vi "Dresden R2R Sputter 03.02.2018 IY24.vi"() -> ()   [LabVIEW 2009] (continued)
                                frame #1 {
                                }
                                }
                                }
                                frame #1 {
                                n15923 = local read "Semi"() -> (w27844)
                                n15924 = case shown="False" w27844 {
                                frame #0 {
                                n15925 = local write "Ch1_PA15"(T/1 ("PA3")) -> ()
                                n15926 = Wait Until Next ms Multiple(millisecond multiple=i32? 1000) -> ()  [unwired: 1 out]
                                }
                                frame #1 {
                                }
                                }
                                }
                                }
                              }
                              frame #1 {
                              }
                            }
                          }
                          frame #10 {
                            # "OPEN CH1-VBV"
                            n15927 = local read "Semi"() -> (w27847)
                            n15928 = case shown="False" w27847 {
                              frame #0 {
                                n15929 = stacked-sequence {
                                frame #0 {
                                n15930 = local read "Semi"() -> (w27848)
                                n15931 = case shown="False" w27848 {
                                frame #0 {
                                n15932 = while {
                                i -> [w27855]
                                stop <- w27850 stop-if-true
                                n15933 = Greater?(x=w27855, y=i32? 50) -> (0:w27853)
                                n15934 = case shown="True" w27853 {
                                frame #0 {
                                }
                                frame #1 {
                                n15935 = local write "Semi"(T/1 ("Semi")) -> ()
                                n15936 = local write "Error Message"("Start up process  cancelled\nbecause  CH1-VBV not opened.\nPlease check  CH1-VBV connections." ("Error Message")) -> ()
                                }
                                }
                                n15937 = local read "Ch1_Ch_atm_di"() -> (w27849)
                                n15938 = case shown="False" w27849 {
                                tunnel: [w27856 T/1] -> w27852
                                frame #0 {
                                n15939 = local read "Ch1_Ch_vbv_di"() -> (w27857)
                                n15940 = case shown="False" w27857 {
                                tunnel: [i16? 0 T/1] -> w27856
                                frame #0 {
                                n15941 = local write "Ch1_Ch_vbv_do"(T/1 ("Ch1_Tp_bv_do")) -> ()
                                n15942 = Wait Until Next ms Multiple(millisecond multiple=i32? 200) -> ()  [unwired: 1 out]
                                }
                                frame #1 {
                                }
                                }
                                }
                                frame #1 {
                                }
                                }
                                n15943 = local read "Semi"() -> (w27851)
                                n15944 = Or(x=w27852, y=w27851) -> (x .or. y?=w27850)
                                }
                                }
                                frame #1 {
                                }
                                }
                                }
                                frame #1 {
                                n15945 = local read "Semi"() -> (w27865)
                                n15946 = case shown="False" w27865 {
                                frame #0 {
                                n15947 = local write "Ch1_PA16"(T/1 ("PA3")) -> ()
                                n15948 = Wait Until Next ms Multiple(millisecond multiple=i32? 1000) -> ()  [unwired: 1 out]
                                }
                                frame #1 {
                                }
                                }
                                }
                                }
                              }
                              frame #1 {
                              }
                            }
                          }
                          frame #11 {
                            # "OPEN/CLOSE TRNS GV-BP2"
                            n15949 = local read "Semi"() -> (w27868)
                            n15950 = case shown="False" w27868 {
                              frame #0 {
                                n15951 = stacked-sequence {
                                frame #0 {
                                n15952 = local read "Semi"() -> (w27869)
                                n15953 = case shown="False" w27869 {
                                frame #0 {
                                n15954 = while {
                                i -> [w27878]
                                stop <- w27873 stop-if-true
                                n15955 = Greater?(x=w27878, y=i32? 800) -> (0:w27876)
                                n15956 = case shown="True" w27876 {
                                frame #0 {
                                }
                                frame #1 {
                                n15957 = local read "Ch2_pressure"() -> (w27898)
                                n15958 = Less?(x=w27898, y=i32? 1) -> (x < y?=w27897)
                                n15959 = case shown="False" w27897 {
                                frame #0 {
                                n15960 = local write "Error Message"("Start up process  cancelled\nbecause  Trns GV-BP2\n not closed.\nPlease check \nTrns GV-BP2 connections." ("Error Message")) -> ()
                                }
                                frame #1 {
                                n15961 = local write "Error Message"("Start up process  cancelled\nbecause  Trns GV-BP2 not\n opened.\nPlease check \nTrns GV-BP2 connections." ("Error Message")) -> ()
                                }
                                }
                                n15962 = local write "Semi"(T/1 ("Semi")) -> ()
                                }
                                }
                                n15963 = local read "Ch2_pressure"() -> (w27872)
                                n15964 = Less?(x=w27872, y=i32? 1) -> (x < y?=w27870)
                                n15965 = case shown="True" w27870 {
                                tunnel: [w27880 w27888] -> w27875
                                frame #0 {
                                n15966 = local read "Ch1_Trns_gv_bp2_di"() -> (w27879)
                                n15967 = case shown="True" w27879 {
                                tunnel: [T/1 i16? 0] -> w27880
                                frame #0 {
                                }
                                frame #1 {
                                n15968 = local write "Ch1_Trns_gv_bp2_do"(i16? 0 ("Ch1_Tp_bv_do")) -> ()
                                n15969 = Wait Until Next ms Multiple(millisecond multiple=i32? 200) -> ()  [unwired: 1 out]
                                }
                                }
                                }
                                frame #1 {
                                n15970 = local read "Ch1_pressure"() -> (w27886)
                                n15971 = Greater Or Equal?(x=w27886, y=dbl? 700.0) -> (x >= y?=w27885)
                                n15972 = case shown="True" w27885 {
                                tunnel: [i16? 0 w27892] -> w27888
                                frame #0 {
                                n15973 = Wait Until Next ms Multiple(millisecond multiple=i32? 500) -> ()  [unwired: 1 out]
                                }
                                frame #1 {
                                n15974 = local read "Ch1_Trns_gv_bp2_di"() -> (w27891)
                                n15975 = case shown="False" w27891 {
                                tunnel: [i16? 0 T/1] -> w27892
                                frame #0 {
                                n15976 = local write "Ch1_Trns_gv_bp2_do"(T/1 ("Ch1_Tp_bv_do")) -> ()
                                n15977 = Wait Until Next ms Multiple(millisecond multiple=i32? 200) -> ()  [unwired: 1 out]
                                }
                                frame #1 {
                                }
                                }
                                }
                                }
                                }
                                }
                                n15978 = local read "Semi"() -> (w27874)
                                n15979 = Or(x=w27875, y=w27874) -> (x .or. y?=w27873)
                                }
                                }
                                frame #1 {
                                }
                                }
                                }
                                frame #1 {
                                n15980 = local read "Semi"() -> (w27903)
                                n15981 = case shown="False" w27903 {
                                frame #0 {
                                n15982 = local write "Ch1_PA17"(T/1 ("PA3")) -> ()
                                n15983 = Wait Until Next ms Multiple(millisecond multiple=i32? 1000) -> ()  [unwired: 1 out]
                                }
                                frame #1 {
                                }
                                }
                                }
                                }
                              }
                              frame #1 {
                              }
                            }
                          }
                          frame #12 {
                            # "CHECK CH-ATM"
                            n15984 = local read "Semi"() -> (w27906)
                            n15985 = case shown="False" w27906 {
                              frame #0 {
                                n15986 = stacked-sequence {
                                frame #0 {
                                n15987 = local read "Semi"() -> (w27907)
                                n15988 = case shown="False" w27907 {
                                frame #0 {
                                n15989 = while {
                                i -> [w27914]
                                stop <- w27909 stop-if-true
                                n15990 = Greater?(x=w27914, y=i32? 1200) -> (0:w27912)
                                n15991 = case shown="True" w27912 {
                                frame #0 {
                                }
                                frame #1 {
                                n15992 = local write "Semi"(T/1 ("Semi")) -> ()
                                n15993 = local write "Error Message"("Start up process  cancelled\nbecause  CH-ATM not opened.\nPlease check CH-ATM connections." ("Error Message")) -> ()
                                }
                                }
                                n15994 = local read "Ch1_Ch_atm_di"() -> (w27908)
                                n15995 = case shown="False" w27908 {
                                tunnel: [i16? 0 T/1] -> w27911
                                frame #0 {
                                n15996 = Wait Until Next ms Multiple(millisecond multiple=i32? 500) -> ()  [unwired: 1 out]
                                }
                                frame #1 {
                                }
                                }
                                n15997 = local read "Semi"() -> (w27910)
                                n15998 = Or(x=w27911, y=w27910) -> (x .or. y?=w27909)
                                }
                                }
                                frame #1 {
                                }
                                }
                                }
                                frame #1 {
                                n15999 = local read "Semi"() -> (w27920)
                                n16000 = case shown="False" w27920 {
                                frame #0 {
                                n16001 = local write "Ch1_PA18"(T/1 ("PA3")) -> ()
                                n16002 = Wait Until Next ms Multiple(millisecond multiple=i32? 1000) -> ()  [unwired: 1 out]
                                }
                                frame #1 {
                                }
                                }
                                }
                                }
                              }
                              frame #1 {
                              }
                            }
                          }
                          frame #13 {
                            # "CLOSE CH1-VBV"
                            n16003 = local read "Semi"() -> (w27923)
                            n16004 = case shown="False" w27923 {
                              frame #0 {
                                n16005 = stacked-sequence {
                                frame #0 {
                                n16006 = local read "Semi"() -> (w27924)
                                n16007 = case shown="False" w27924 {
                                frame #0 {
                                n16008 = while {
                                i -> [w27931]
                                stop <- w27925 stop-if-true
                                n16009 = Greater?(x=w27931, y=i32? 50) -> (0:w27929)
                                n16010 = case shown="True" w27929 {
                                frame #0 {
                                }
                                frame #1 {
                                n16011 = local write "Semi"(T/1 ("Semi")) -> ()
                                n16012 = local write "Error Message"("Start up process  cancelled\nbecause  CH1-VBV not closed.\nPlease check  CH1-VBV connections." ("Error Message")) -> ()
                                }
                                }
                                n16013 = local read "Ch1_Ch_vbv_di"() -> (w27928)
                                n16014 = case shown="True" w27928 {
                                tunnel: [T/1 i16? 0] -> w27927
                                frame #0 {
                                }
                                frame #1 {
                                n16015 = Wait Until Next ms Multiple(millisecond multiple=i32? 200) -> ()  [unwired: 1 out]
                                n16016 = local write "Ch1_Ch_vbv_do"(i16? 0 ("Ch1_Tp_bv_do")) -> ()
                                }
                                }
                                n16017 = local read "Semi"() -> (w27926)
                                n16018 = Or(x=w27927, y=w27926) -> (x .or. y?=w27925)
                                }
                                }
                                frame #1 {
                                }
                                }
                                }
                                frame #1 {
                                n16019 = local read "Semi"() -> (w27938)
                                n16020 = case shown="False" w27938 {
                                frame #0 {
                                n16021 = local write "Ch1_PA19"(T/1 ("PA3")) -> ()
                                n16022 = Wait Until Next ms Multiple(millisecond multiple=i32? 1000) -> ()  [unwired: 1 out]
                                }
                                frame #1 {
                                }
                                }
                                }
                                }
                              }
                              frame #1 {
                              }
                            }
                          }
                          frame #14 {
                            # "Close PL-VBV"
                            n16023 = local read "Semi"() -> (w27941)
                            n16024 = case shown="False" w27941 {
                              frame #0 {
                                n16025 = stacked-sequence {
                                frame #0 {
                                n16026 = local read "Semi"() -> (w27942)
                                n16027 = case shown="False" w27942 {
                                frame #0 {
                                n16028 = while {
                                i -> [w27949]
                                stop <- w27943 stop-if-true
                                n16029 = Greater?(x=w27949, y=i32? 50) -> (0:w27947)
                                n16030 = case shown="True" w27947 {
                                frame #0 {
                                }
                                frame #1 {
                                n16031 = local write "Semi"(T/1 ("Semi")) -> ()
                                n16032 = local write "Error Message"("Start up process  cancelled\nbecause  PL1-VBV not closed.\nPlease check PL1-VBV connections." ("Error Message")) -> ()
                                }
                                }
                                n16033 = local read "Ch1_Pl_vbv_di"() -> (w27946)
                                n16034 = case shown="True" w27946 {
                                tunnel: [T/1 i16? 0] -> w27945
                                frame #0 {
                                }
                                frame #1 {
                                n16035 = Wait Until Next ms Multiple(millisecond multiple=i32? 200) -> ()  [unwired: 1 out]
                                n16036 = local write "Ch1_Pl_vbv_do"(i16? 0 ("Ch1_Tp_bv_do")) -> ()
                                }
                                }
                                n16037 = local read "Semi"() -> (w27944)
                                n16038 = Or(x=w27945, y=w27944) -> (x .or. y?=w27943)
                                }
                                }
                                frame #1 {
                                }
                                }
                                }
                                frame #1 {
                                n16039 = local read "Semi"() -> (w27956)
                                n16040 = case shown="False" w27956 {
                                frame #0 {
                                n16041 = local write "Ch1_PA20"(T/1 ("PA3")) -> ()
                                n16042 = Wait Until Next ms Multiple(millisecond multiple=i32? 1000) -> ()  [unwired: 1 out]
                                }
                                frame #1 {
                                }
                                }
                                }
                                }
                              }
                              frame #1 {
                              }
                            }
                          }
                          frame #15 {
                            # "OPEN TP-BV"
                            n16043 = local read "Semi"() -> (w27959)
                            n16044 = case shown="False" w27959 {
                              frame #0 {
                                n16045 = stacked-sequence {
                                frame #0 {
                                n16046 = local read "Semi"() -> (w27960)
                                n16047 = case shown="False" w27960 {
                                frame #0 {
                                n16048 = while {
                                i -> [w27967]
                                stop <- w27962 stop-if-true
                                n16049 = Greater?(x=w27967, y=i32? 50) -> (0:w27965)
                                n16050 = case shown="True" w27965 {
                                frame #0 {
                                }
                                frame #1 {
                                n16051 = local write "Semi"(T/1 ("Semi")) -> ()
                                n16052 = local write "Error Message"("Start up process  cancelled\nbecause  TP-BV not opened.\nPlease check TP-BV1 connections." ("Error Message")) -> ()
                                }
                                }
                                n16053 = local read "Ch1_Tp_bv_di"() -> (w27961)
                                n16054 = case shown="False" w27961 {
                                tunnel: [i16? 0 T/1] -> w27964
                                frame #0 {
                                n16055 = Wait Until Next ms Multiple(millisecond multiple=i32? 200) -> ()  [unwired: 1 out]
                                n16056 = local write "Ch1_Tp_bv_do"(T/1 ("Ch1_Tp_bv_do")) -> ()
                                }
                                frame #1 {
                                }
                                }
                                n16057 = local read "Semi"() -> (w27963)
                                n16058 = Or(x=w27964, y=w27963) -> (x .or. y?=w27962)
                                }
                                }
                                frame #1 {
                                }
                                }
                                }
                                frame #1 {
                                n16059 = local read "Semi"() -> (w27974)
                                n16060 = case shown="False" w27974 {
                                frame #0 {
                                n16061 = local write "Ch1_PA21"(T/1 ("PA3")) -> ()
                                n16062 = Wait Until Next ms Multiple(millisecond multiple=i32? 1000) -> ()  [unwired: 1 out]
                                }
                                frame #1 {
                                }
                                }
                                }
                                }
                              }
                              frame #1 {
                              }
                            }
                          }
                          frame #16 {
                            # "CLOSE CH1-ATM"
                            n16063 = local read "Semi"() -> (w27977)
                            n16064 = case shown="False" w27977 {
                              frame #0 {
                                n16065 = stacked-sequence {
                                frame #0 {
                                n16066 = local read "Semi"() -> (w27978)
                                n16067 = case shown="False" w27978 {
                                frame #0 {
                                n16068 = while {
                                i -> [w27985]
                                stop <- w27979 stop-if-true
                                n16069 = Greater?(x=w27985, y=i32? 50) -> (0:w27983)
                                n16070 = case shown="True" w27983 {
                                frame #0 {
                                }
                                frame #1 {
                                n16071 = local write "Semi"(T/1 ("Semi")) -> ()
                                n16072 = local write "Error Message"("Start up process  cancelled\nbecause CH1-ATM not closed.\nPlease check CH1-ATM connections." ("Error Message")) -> ()
                                }
                                }
                                n16073 = local read "Ch1_Ch_atm_di"() -> (w27982)
                                n16074 = case shown="True" w27982 {
                                tunnel: [T/1 i16? 0] -> w27981
                                frame #0 {
                                }
                                frame #1 {
                                n16075 = Wait Until Next ms Multiple(millisecond multiple=i32? 200) -> ()  [unwired: 1 out]
                                n16076 = local write "Ch1_Ch_atm_do"(T/1 ("Ch1_Tp_bv_do")) -> ()
                                }
                                }
                                n16077 = local read "Semi"() -> (w27980)
                                n16078 = Or(x=w27981, y=w27980) -> (x .or. y?=w27979)
                                }
                                }
                                frame #1 {
                                }
                                }
                                }
                                frame #1 {
                                n16079 = local read "Semi"() -> (w27992)
                                n16080 = case shown="False" w27992 {
                                frame #0 {
                                n16081 = local write "Ch1_PA22"(T/1 ("PA3")) -> ()
                                n16082 = Wait Until Next ms Multiple(millisecond multiple=i32? 1000) -> ()  [unwired: 1 out]
                                }
                                frame #1 {
                                }
                                }
                                }
                                }
                              }
                              frame #1 {
                              }
                            }
                          }
                          frame #17 {
                            # "CLOSE PL1-ATM"
                            n16083 = local read "Semi"() -> (w27995)
                            n16084 = case shown="False" w27995 {
                              frame #0 {
                                n16085 = stacked-sequence {
                                frame #0 {
                                n16086 = local read "Semi"() -> (w27996)
                                n16087 = case shown="False" w27996 {
                                frame #0 {
                                n16088 = while {
                                i -> [w28003]
                                stop <- w27997 stop-if-true
                                n16089 = Greater?(x=w28003, y=i32? 50) -> (0:w28001)
                                n16090 = case shown="True" w28001 {
                                frame #0 {
                                }
                                frame #1 {
                                n16091 = local write "Semi"(T/1 ("Semi")) -> ()
                                n16092 = local write "Error Message"("Start up process  cancelled\nbecause  PL-ATM not closed.\nPlease check PL-ATM1 connections." ("Error Message")) -> ()
                                }
                                }
                                n16093 = local read "Ch1_Pl_atm_di"() -> (w28000)
                                n16094 = case shown="True" w28000 {
                                tunnel: [T/1 i16? 0] -> w27999
                                frame #0 {
                                }
                                frame #1 {
                                n16095 = Wait Until Next ms Multiple(millisecond multiple=i32? 200) -> ()  [unwired: 1 out]
                                n16096 = local write "Ch1_Pl_atm_do"(T/1 ("Ch1_Tp_bv_do")) -> ()
                                }
                                }
                                n16097 = local read "Semi"() -> (w27998)
                                n16098 = Or(x=w27999, y=w27998) -> (x .or. y?=w27997)
                                }
                                }
                                frame #1 {
                                }
                                }
                                }
                                frame #1 {
                                n16099 = local read "Semi"() -> (w28010)
                                n16100 = case shown="False" w28010 {
                                frame #0 {
                                n16101 = local write "Ch1_PA23"(T/1 ("PA3")) -> ()
                                n16102 = Wait Until Next ms Multiple(millisecond multiple=i32? 1000) -> ()  [unwired: 1 out]
                                }
                                frame #1 {
                                }
                                }
                                }
                                }
                              }
                              frame #1 {
                              }
                            }
                          }
                          frame #18 {
                            # "START MP"
                            n16103 = local read "Semi"() -> (w28013)
                            n16104 = case shown="False" w28013 {
                              frame #0 {
                                n16105 = stacked-sequence {
                                frame #0 {
                                n16106 = local read "Semi"() -> (w28014)
                                n16107 = case shown="False" w28014 {
                                frame #0 {
                                n16108 = while {
                                i -> [w28021]
                                stop <- w28015 stop-if-true
                                n16109 = Greater?(x=w28021, y=i32? 50) -> (0:w28019)
                                n16110 = case shown="True" w28019 {
                                frame #0 {
                                }
                                frame #1 {
                                n16111 = local write "Semi"(T/1 ("Semi")) -> ()
                                n16112 = local write "Error Message"("Start up process  cancelled\nbecause MP1 not started.\nPlease check MP1 connections." ("Error Message")) -> ()
                                }
                                }
                                n16113 = local read "Ch1_Mp_di"() -> (w28018)
                                n16114 = case shown="False" w28018 {
                                tunnel: [i16? 0 T/1] -> w28017
                                frame #0 {
                                n16115 = Wait Until Next ms Multiple(millisecond multiple=i32? 200) -> ()  [unwired: 1 out]
                                n16116 = local write "Ch1_Mp_do"(T/1 ("Ch1_Tp_bv_do")) -> ()
                                }
                                frame #1 {
                                }
                                }
                                n16117 = local read "Semi"() -> (w28016)
                                n16118 = Or(x=w28017, y=w28016) -> (x .or. y?=w28015)
                                }
                                }
                                frame #1 {
                                }
                                }
                                }
                                frame #1 {
                                n16119 = local read "Semi"() -> (w28028)
                                n16120 = case shown="False" w28028 {
                                frame #0 {
                                n16121 = local write "Ch1_PA24"(T/1 ("PA3")) -> ()
                                n16122 = Wait Until Next ms Multiple(millisecond multiple=i32? 1000) -> ()  [unwired: 1 out]
                                }
                                frame #1 {
                                }
                                }
                                }
                                }
                              }
                              frame #1 {
                              }
                            }
                          }
                          frame #19 {
                            # "START TP"
                            n16123 = local read "Semi"() -> (w28031)
                            n16124 = case shown="False" w28031 {
                              frame #0 {
                                n16125 = stacked-sequence {
                                frame #0 {
                                n16126 = local read "Semi"() -> (w28032)
                                n16127 = case shown="False" w28032 {
                                frame #0 {
                                n16128 = stacked-sequence {
                                frame #0 {
                                n16129 = local read "Semi"() -> (w28033)
                                n16130 = case shown="False" w28033 {
                                frame #0 {
                                n16131 = local write "Tp1_auto_start"(T/1 ("Tp1_auto_start")) -> ()
                                }
                                frame #1 {
                                }
                                }
                                }
                                frame #1 {
                                n16132 = local read "Semi"() -> (w28035)
                                n16133 = case shown="False" w28035 {
                                frame #0 {
                                n16134 = Wait (ms)(milliseconds to wait=i32? 1000) -> ()  [unwired: 1 out]
                                }
                                frame #1 {
                                }
                                }
                                }
                                frame #2 {
                                n16135 = local read "Semi"() -> (w28037)
                                n16136 = case shown="False" w28037 {
                                frame #0 {
                                n16137 = local write "Tp1_auto_start"(T/1 ("Tp1_auto_start")) -> ()
                                }
                                frame #1 {
                                }
                                }
                                }
                                }
                                }
                                frame #1 {
                                }
                                }
                                }
                                frame #1 {
                                n16138 = local read "Semi"() -> (w28039)
                                n16139 = case shown="False" w28039 {
                                frame #0 {
                                n16140 = local write "Ch1_PA29"(T/1 ("PA3")) -> ()
                                n16141 = Wait Until Next ms Multiple(millisecond multiple=i32? 1000) -> ()  [unwired: 1 out]
                                }
                                frame #1 {
                                }
                                }
                                }
                                }
                              }
                              frame #1 {
                              }
                            }
                          }
                          frame #20 {
                            # "CHECK PL-PRESSURE"
                            n16142 = local read "Semi"() -> (w28042)
                            n16143 = case shown="False" w28042 {
                              frame #0 {
                                n16144 = stacked-sequence {
                                frame #0 {
                                n16145 = local read "Semi"() -> (w28043)
                                n16146 = case shown="False" w28043 {
                                frame #0 {
                                n16147 = while {
                                i -> [w28052]
                                stop <- w28047 stop-if-true
                                n16148 = Greater?(x=w28052, y=i32? 1200) -> (0:w28050)
                                n16149 = case shown="True" w28050 {
                                frame #0 {
                                }
                                frame #1 {
                                n16150 = local write "Semi"(T/1 ("Semi")) -> ()
                                n16151 = local write "Error Message"("Start up process was cancelled.\nPlease check Pipeline \nvacuum connections." ("Error Message")) -> ()
                                }
                                }
                                n16152 = local read "Pl_pg_press_ch1"() -> (w28046)
                                n16153 = Less?(x=w28046, y=dbl? 0.9) -> (x < y?=w28044)
                                n16154 = case shown="False" w28044 {
                                tunnel: [i16? 0 T/1] -> w28049
                                frame #0 {
                                n16155 = Wait Until Next ms Multiple(millisecond multiple=i32? 500) -> ()  [unwired: 1 out]
                                }
                                frame #1 {
                                }
                                }
                                n16156 = local read "Semi"() -> (w28048)
                                n16157 = Or(x=w28049, y=w28048) -> (x .or. y?=w28047)
                                }
                                }
                                frame #1 {
                                }
                                }
                                }
                                frame #1 {
                                n16158 = local read "Semi"() -> (w28058)
                                n16159 = case shown="False" w28058 {
                                frame #0 {
                                n16160 = local write "Ch1_PA25"(T/1 ("PA3")) -> ()
                                n16161 = Wait Until Next ms Multiple(millisecond multiple=i32? 1000) -> ()  [unwired: 1 out]
                                }
                                frame #1 {
                                }
                                }
                                }
                                }
                              }
                              frame #1 {
                              }
                            }
                          }
                          frame #21 {
                            # "CHECK CH-PRESSURE"
                            n16162 = local read "Semi"() -> (w28061)
                            n16163 = case shown="False" w28061 {
                              frame #0 {
                                n16164 = stacked-sequence {
                                frame #0 {
                                n16165 = local read "Semi"() -> (w28062)
                                n16166 = case shown="False" w28062 {
                                frame #0 {
                                n16167 = while {
                                i -> [w28071]
                                stop <- w28066 stop-if-true
                                n16168 = Greater?(x=w28071, y=i32? 1200) -> (0:w28069)
                                n16169 = case shown="True" w28069 {
                                frame #0 {
                                }
                                frame #1 {
                                n16170 = local write "Semi"(T/1 ("Semi")) -> ()
                                n16171 = local write "Error Message"("Start up process was cancelled.\nPlease check chamber \nvacuum connections." ("Error Message")) -> ()
                                }
                                }
                                n16172 = local read "Ch1_pressure"() -> (w28065)
                                n16173 = Less?(x=w28065, y=dbl? 0.9) -> (x < y?=w28063)
                                n16174 = case shown="False" w28063 {
                                tunnel: [i16? 0 T/1] -> w28068
                                frame #0 {
                                n16175 = Wait Until Next ms Multiple(millisecond multiple=i32? 500) -> ()  [unwired: 1 out]
                                }
                                frame #1 {
                                }
                                }
                                n16176 = local read "Semi"() -> (w28067)
                                n16177 = Or(x=w28068, y=w28067) -> (x .or. y?=w28066)
                                }
                                }
                                frame #1 {
                                }
                                }
                                }
                                frame #1 {
                                n16178 = local read "Semi"() -> (w28077)
                                n16179 = case shown="False" w28077 {
                                frame #0 {
                                n16180 = local write "Ch1_PA26"(T/1 ("PA3")) -> ()
                                n16181 = Wait Until Next ms Multiple(millisecond multiple=i32? 1000) -> ()  [unwired: 1 out]
                                }
                                frame #1 {
                                }
                                }
                                }
                                }
                              }
                              frame #1 {
                              }
                            }
                          }
                          frame #22 {
                            # "OPEN BG-BV"
                            n16182 = local read "Semi"() -> (w28080)
                            n16183 = case shown="False" w28080 {
                              frame #0 {
                                n16184 = stacked-sequence {
                                frame #0 {
                                n16185 = local read "Semi"() -> (w28081)
                                n16186 = case shown="False" w28081 {
                                frame #0 {
                                n16187 = while {
                                i -> [w28088]
                                stop <- w28083 stop-if-true
                                n16188 = Greater?(x=w28088, y=i32? 50) -> (0:w28086)
                                n16189 = case shown="True" w28086 {
                                frame #0 {
                                }
                                frame #1 {
                                n16190 = local write "Semi"(T/1 ("Semi")) -> ()
                                n16191 = local write "Error Message"("Start up process  cancelled\nbecause  BG-BV not opened.\nPlease check BG-BV1 connections." ("Error Message")) -> ()
                                }
                                }
                                n16192 = local read "Ch1_Bg_bv_di"() -> (w28082)
                                n16193 = case shown="False" w28082 {
                                tunnel: [i16? 0 T/1] -> w28085
                                frame #0 {
                                n16194 = Wait Until Next ms Multiple(millisecond multiple=i32? 200) -> ()  [unwired: 1 out]
                                n16195 = local write "Ch1_Bg_bv_do"(T/1 ("Ch1_Tp_bv_do")) -> ()
                                }
                                frame #1 {
                                }
                                }
                                n16196 = local read "Semi"() -> (w28084)
                                n16197 = Or(x=w28085, y=w28084) -> (x .or. y?=w28083)
                                }
                                }
                                frame #1 {
                                }
                                }
                                }
                                frame #1 {
                                n16198 = local read "Semi"() -> (w28095)
                                n16199 = case shown="False" w28095 {
                                frame #0 {
                                n16200 = local write "Ch1_PA27"(T/1 ("PA3")) -> ()
                                n16201 = Wait Until Next ms Multiple(millisecond multiple=i32? 1000) -> ()  [unwired: 1 out]
                                }
                                frame #1 {
                                }
                                }
                                }
                                }
                              }
                              frame #1 {
                              }
                            }
                          }
                          frame #23 {
                            # "CHECK CH-PRESSURE"
                            n16202 = local read "Semi"() -> (w28098)
                            n16203 = case shown="False" w28098 {
                              frame #0 {
                                n16204 = stacked-sequence {
                                frame #0 {
                                n16205 = local read "Semi"() -> (w28099)
                                n16206 = case shown="False" w28099 {
                                frame #0 {
                                n16207 = while {
                                i -> [w28108]
                                stop <- w28103 stop-if-true
                                n16208 = Greater?(x=w28108, y=i32? 600) -> (0:w28106)
                                n16209 = case shown="True" w28106 {
                                frame #0 {